vi "MPS_main.vi"() -> ()   [LabVIEW 2021]
uses:
  <vilib>/Analysis/4window.llb/windowTd.ctl
  <vilib>/DAQmx/write.llb/DAQmx Write (Digital Bool 1Line 1Point).vi
  <extravilib>/ChannelInstances/Tag-dbl/Write With Abort.vi
  <vilib>/Utility/file.llb/Write Delimited Spreadsheet (DBL).vi
  MPS_global_variables.vi
  <vilib>/DAQmx/create/channels.llb/DAQmx Create Channel (DO-Digital Output).vi
  <vilib>/DAQmx/miscellaneous.llb/DAQmx Fill In Error Info.vi
  <extravilib>/ChannelInstances/Tag-dbl/Instantiate.vi
  <extravilib>/ChannelInstances/Tag-dbl/Endpoint.vi
  <vilib>/measure/maspectr.llb/FFT Spectrum (Mag-Phase) for 1 Chan.vi
  <extravilib>/ChannelInstances/Tag-dbl.lvlib
  <vilib>/measure/NI_MAPro.lvlib
  <vilib>/Analysis/NI_AALPro.lvlib
  <vilib>/Analysis/NI_AALBase.lvlib
  <vilib>/gmath/NI_Gmath.lvlib
panel:
  out "Last N Drive Amp":dbl[](array[numeric])=[7.800948435870364e-05, 7.800948435870364e-05, 7.800948435870364e-05, 7.800948435870364e-05, 7.800948435870364e-05]
  in  "Divide By val":dbl=2.0
  in  "Divide Mass by X":bool
  in  "Zero Baseline":bool
  out "Waveform Graph":dbl[][](graph)
  out "Sensitivity profile 2":dbl[][](graph)
  out "Recent File Name":string="SP_Fill in name_60_ug_Batch Name"
  in  "name identifier":string="Fill in name"
  in  "Base path":path=path "D:/HumanImagerData/MPS Data"
  out "Meas Drive IMon Val RMS\nCal BMon":dbl=16.19447647785509
  in  "Acq Baseline":bool
  in  "CalcConc":bool
  in  "CalcMass":bool
  in  "Sample MetaData Cluster":T1={"Sample Volume (uL)"=10.0, "Sample Mass (ug)"=60.0, "Sample Conc(mg/mL)"=6.0, "Sample Temperature (C)"=23.0, "Batch Num"=0.0, "Batch Name"="Batch Name", "Solute"="Fe3O4", "Solvent"="Water ", "Sample Description"="Description"}
  in  "TxRx_Params":T2={"sample rate"=2000000.0, "Tx freq"=23809.52380952381, "Tx amp"=0.95, "Tx cycles\nSpectroscopy"=250.0, "Bias amp"=1.4, "Bias freq"=11.904761904761905, "Receive range"=5.0, "Bias Periods\nMagnetometry"=2.0, "Tx Freq Division Factor"=84.0, "Drive Periods per Bias"=2000.0, "TX harmonics"=[47619.04761904762, 71428.57142857142, 95238.09523809524, 119047.61904761905, 142857.14285714284, 166666.66666666666, 190476.19047619047, 214285.7142857143, 238095.2380952381, 261904.7619047619, 285714.2857142857, 309523.8095238095, 333333.3333333333, 357142.85714285716, 380952.38095238095, 404761.90476190473, 428571.4285714286, 452380.95238095237, 476190.4761904762, 500000.0, 523809.5238095238, 547619.0476190476, 571428.5714285714, 595238.0952380953, 619047.619047619, 642857.1428571428, 666666.6666666666, 690476.1904761904, 714285.7142857143, 738095.2380952381, 761904.7619047619, 785714.2857142857, 809523.8095238095, 833333.3333333334, 857142.8571428572, 880952.380952381, 904761.9047619047, 928571.4285714285]} {"TX harmonics" format="%#_6p"; "Tx freq" format="%#_8g"}
  in  "Tab Control 2":enum32{"Motor Params", "Motor Move Control"}(tab)=enum."Motor Move Control"
  out "Motor Dir\nT=Fwd":bool=TRUE
  in  "pulse duration (T/2)":dbl=0.0005 format="%#_13p"
  in  "Motor speed":string(combo)="Full step"
  in  "Sequence to run on start up":string[](array[string])=["Move", "Halt"]
  out "Current Motor State":string="MoveToMax"
  in  "Unsigned Pulses to move":dbl=10.0
  in  "Move-Bed-Back":bool
  in  "Move-Bed-Fwd":bool
  in  "Home then insert sample":bool
  in  "Pulses From Home to Max Sig":dbl=4400.0
  in  "Motor Go Home":bool
  in  "Pulses to move fwd after homing":dbl=150.0 format="%#_13g"
  out "Empty Bore-BMon-Spec":dbl[](array[numeric])
  out "EmptyBoreBaseline_Mag_BMon":dbl[](array[numeric])
  in  "Toggle fan":bool
  out "Amps Drive Peak":dbl=22.902448270514743 format="%#_3p"
  out "EmptyBoreBaseline_Mag":dbl[](array[numeric])
  out "Samples Per Acquisition":dbl=336000.0
  in  "Run Cal BMon":bool
  out "mT/BMon Volt":dbl=145.27846134703603 format="%#_3p"
  out "Meas BMon Val RMS":dbl=0.11147197132801606 format="%#_3p"
  out "Expected mT peak":dbl=10.428171771013478 format="%#_3p"
  in  "Update global variables Button":bool
  in  "stop":bool
  out "current system state":string="Idle"
  out "Main loop has stopped":bool
  in  "Tab Control":T3(tab)
  in  "Tab Control 3":enum32{"Page 1", "Page 2"}(tab)=enum."Page 2"
  out "Mean of mags TF Corr":dbl[](array[numeric])=[4.5198134161737477e-10, 4.705339091228016e-11, 2.4913628541095572e-11, 3.799080385209649e-11, 3.684657264994396e-11, 2.7666013040822994e-11, 2.1562998262072176e-11, 9.35832283593572e-12, 6.785335767128005e-12, 1.618637654777638e-11, 4.453278972759378e-12, 8.695242161562175e-12, 5.505695421570372e-12, 7.599580036290615e-12, 4.816377102414867e-12, 1.3029297120510833e-12, 1.361107900144818e-12, 1.5509807531885633e-13, 1.1494126125683072e-12, 1.8048572256788235e-12, 1.5695940756056345e-12, 4.177554610240691e-12, 5.999424509842453e-12, 4.874978557021519e-12, 9.529122987805845e-12, 5.379691887303521e-12, 9.75617748882951e-12, 1.0753597956189388e-11, 1.383578141946564e-11, 1.3802076818093284e-11, 1.2509628346279071e-11, 1.7443696397243005e-11, 1.9010656363318516e-11, 2.256704924965476e-11, 3.9887752269893355e-11, 3.312089204703278e-11, 2.9142643692279936e-11, 4.5578886589904716e-11, 2.966185216911441e-11, 0.0] format="%#_3p"
  out "mean(FFT) mag":cluster{"Freq array":dbl[], dbl[]}[](graph)
  out "std(FFT)":cluster{"Freq array":dbl[], dbl[]}[](graph)
  out "Std of mags TF Corr":dbl[](array[numeric])=[2.4765666807740003e-10, 2.964765473975954e-11, 1.8138460819953634e-11, 1.2295124978270651e-11, 8.877087369588469e-12, 9.76692294864142e-12, 1.1060107857364228e-11, 5.4800226806312794e-12, 3.1400058412540406e-12, 6.864203903815931e-12, 2.747684195772991e-12, 3.0948587149085473e-12, 2.32071663594191e-12, 2.4779399251558228e-12, 1.8375422203984164e-12, 9.224659898036068e-13, 6.04641015605487e-13, 7.10975452417779e-14, 4.585024773080199e-13, 4.784974514194064e-13, 1.0687637252520008e-12, 1.6948060875352746e-12, 2.7148006011093817e-12, 2.5718695170368923e-12, 4.860185837662061e-12, 2.2698952232635406e-12, 2.837534889875566e-12, 6.3680645161241505e-12, 5.393413394622827e-12, 3.866615680263908e-12, 4.896578402975936e-12, 1.0408434178007631e-11, 1.1521799342350357e-11, 1.2111931519408025e-11, 2.1261630231843856e-11, 2.1498039397344003e-11, 1.6468567943662256e-11, 1.9206279692837516e-11, 1.6162742557341904e-11, 0.0] format="%#_3p"
  out "mean(FFT) Tx Current":cluster{"Freq array":dbl[], dbl[]}(graph)
  out "std(FFT)  Tx Current":cluster{"Freq array":dbl[], dbl[]}(graph)
  in  "Run Sys Ref Meas":bool
  in  "Save SRM":bool
  in  "Spec Tx periods\nto crop SRM":dbl=150.0 format="%#_4p"
  in  "ms delay SRM":u32=5 format="%#.4p"
  in  "Num Avgs SRM":i32=10
  in  "Apply drift \ncorrection?":bool=TRUE
  out "size(s)":i32=4200 format="%.0p"
  out "Loop Num 3":i32=9
  out "Mean_IMon_THD":dbl=0.011152455970515396 format="%#_3p"
  out "MeanIMonTHD_dB":dbl=-39.052589653230974 format="%#_3p"
  in  "Scanner Description":T4={"Scanner Name"="MGH_MIT_MPS", "Hardware description"="Test", "Preamplifier Used"="INA", "Preamp Gain"=9999.0, "Drive Amplifier"="RCF IPS700_CH1", "Bias Amplifier"="RCF IPS700_CH2", "Drive Current Monitor"="Rogowski", "Bias Current Monitor"="ACS-770"}
  in  "Study and Experiment Description":T5={"Study Number"=1, "Study Name"="Particle Testing", "UUID"="B5C626AE-1F0E-494D-B0C0-DF45A2631BD1", "GUI Open Time"="2023-07-01_12-07-36", "Notes"="Dilution Series"}
  out "3f0 over time":cluster{dbl, dbl}(graph)={9.606056730162145e-13, 8.787008379959242e-12}
  out "Rx FFT":cluster{"f0":dbl, "df":dbl, "magnitude":dbl[]}(graph)={"f0"=0.0, "df"=158.7301587301721, "magnitude"=array[6300 elements]}
  in  "Run Spectroscopy":bool
  in  "Stop Spec":bool
  out "Loop Num":i32=9 format="%#.3p"
  in  "Save Spectroscopy":bool
  in  "Max Spec Runs":i32=500
  in  "ms delay":u32=1 format="%#.4p"
  in  "Spec Tx periods\nto crop":dbl=100.0 format="%#_4p"
  out "Spec Time Domain":waveform(dbl)[](graph)=[{"t0"=timestamp(3771075099.535634 s since 1904-01-01), "dt"=4.999999999999579e-07, "Y"=array[159600 elements], "attributes"=variant("NI_ChannelName"=variant(string "H1/ai7"), "NI_UnitDescription"=variant(string "Volts"))}, {"t0"=timestamp(3771075099.535634 s since 1904-01-01), "dt"=4.999999999999579e-07, "Y"=array[159600 elements], "attributes"=variant("NI_ChannelName"=variant(string "H1/ai7"), "NI_UnitDescription"=variant(string "Volts"))}, {"t0"=timestamp(3771075099.535634 s since 1904-01-01), "dt"=4.999999999999579e-07, "Y"=array[159600 elements], "attributes"=variant("NI_ChannelName"=variant(string "H1/ai7"), "NI_UnitDescription"=variant(string "Volts"))}]
  out "f0 over time":dbl(graph)=1.7007410257248368e-10
  out "THD":dbl=0.005520776982623166 format="%#_4p"
  out "Expected mT Spec Drive":dbl=6.10435204788981e-05 format="%#_4p"
  out "mean3f0":dbl=3.4713942019657602e-12 format="%#_3p"
  out "standard deviation 3f0":dbl=1.6525895136355058e-12 format="%#_4p"
  out "meanf0":dbl=1.0516138967766213e-10 format="%#_3p"
  out "standard deviation f0":dbl=4.090729980375604e-11 format="%#_4p"
  out "Ref mT Spec Drive":dbl=7.800948435870364e-05 format="%#_4p"
  in  "UseFeedback":bool
  out "f0 Phase over time":dbl(graph)=-0.927647026653393
  in  "Feedback Avging":dbl=5.0 format="%#_13g"
  out "Relative mT Drive":dbl=0.00016343259278743684 format="%#_3p"
  out "Updated Tx Amp":dbl=0.5023739790026548
  out "Error":dbl=0.0016712299166545819 format="%#_3p"
  in  "Error Gain":dbl=0.1
  out "Langevin":cluster{"Y":dbl[], "Y":dbl[]}[](graph)=[{"Y"=[-3.899866061425817e-05, -3.9231748974479236e-05, -3.9246824870256426e-05, -3.904388830702801e-05, -3.8622939290039456e-05, -3.798845753237372e-05, -3.714641598259823e-05, -3.609830788135816e-05, -3.484562646899217e-05, -3.3398824400567615e-05, -3.17653678589874e-05, -2.9952723026593753e-05, -2.7975822263882995e-05, -2.584511822356924e-05, -2.3569570322071078e-05, -2.1164110918043826e-05, -1.8640685898287753e-05, -1.6012734384739088e-05, -1.3296681970143925e-05, -1.0508954246793974e-05, -7.66448357105398e-06, -4.776709063440463e-06, -1.8620563154459617e-06, 1.0585693748465211e-06, 3.971728887269857e-06, 6.863983101619107e-06, 9.714426719695402e-06, 1.2511113856608338e-05, 1.5237618920418202e-05, 1.7876023083287668e-05, 2.0415873695016075e-05, 2.284223839813179e-05, 2.5137198363318037e-05, 2.7290300939033318e-05, 2.9291093473156727e-05, 3.1124643605919247e-05, 3.278199191982424e-05, 3.425268576098663e-05, 3.553224541833137e-05, 3.661320470851545e-05, 3.7486604212060796e-05, 3.815244392424258e-05, 3.8606244132429925e-05, 3.8842031887654564e-05, 3.885831394862594e-05, 3.8658076782053854e-05, 3.824132038257107e-05, 3.760655150867529e-05, 3.6758249863472383e-05, 3.5703881622719267e-05, 3.444941972643954e-05, 3.300233035134814e-05, 3.1368586438269434e-05, 2.9558640637570703e-05, 2.7584438836498958e-05, 2.545494045026684e-05, 2.3176118421620688e-05, 2.0765891585527157e-05, 1.8246658487001164e-05, 1.5625885307065433e-05, 1.2912531463566184e-05, 1.0126009030398355e-05, 7.282743608825543e-06, 4.3961743274289376e-06, 1.4857132611988467e-06, -1.4337072243640028e-06, -4.3471547637050135e-06, -7.236710518203559e-06, -1.0085948885939363e-05, -1.2881430738303868e-05, -1.560374400091777e-05, -1.8239449545843204e-05, -2.077809471867073e-05, -2.3203253919419743e-05, -2.5499994785286915e-05, -2.7654878190523024e-05, -2.9655958246518067e-05, -3.148979582892112e-05, -3.314892475944235e-05, -3.462438562405869e-05, -3.5905725772938516e-05, -3.69869722656569e-05, -3.786364539834503e-05, -3.853126546745361e-05], "Y"=[5.7665139055820235e-05, 8.02563342374943e-05, 2.3135954141162975e-05, 3.8370395851491655e-05, 7.666887421492822e-08, -1.6353326745701167e-06, -3.131850109735249e-05, -4.252180215784362e-05, -6.681075201303612e-05, -8.354178500796668e-05, -0.00011232913710735343, -0.00011212036199780602, -0.00015658876280484033, -0.0001388647952584951, -0.0001842459865776697, -0.00017643225669247359, -0.00020075124710503323, -0.00020291853502768815, -0.00021791460296951315, -0.00021365035373967857, -0.00023303765092765828, -0.0002161064064262681, -0.0002478914872234107, -0.00022194556056100495, -0.00024165239405261733, -0.00022831141293448037, -0.00023730193869174858, -0.0002282319404163689, -0.00022891465369582039, -0.00022086199509847537, -0.00021075781792146404, -0.00019855575075151182, -0.0001986104750695162, -0.0001784588780601685, -0.00018112303600478357, -0.00018159513469144167, -0.0001503133846049755, -0.00017229903149902393, -0.00012674935866696186, -0.0001344447370080244, -0.00010040371918754682, -0.0001009590608068881, -8.558721246688338e-05, -6.95419396555478e-05, -6.45994581417109e-05, -3.476218814891166e-05, -2.3990356126791314e-05, 1.1960562969286733e-05, 1.1320497334370813e-05, 6.587790071654025e-05, 4.0726279326073945e-05, 8.901605718512913e-05, 8.626069687517241e-05, 8.544329637751575e-05, 0.000135062345200515, 0.00010999614741809734, 0.0001695727606417653, 0.00015403057543677463, 0.0001959948576704691, 0.00017327275872732083, 0.00020990531288118922, 0.0001997518664420034, 0.0002049616944248637, 0.00023545186254814868, 0.00022864323236331527, 0.000242514729569909, 0.00024575451950278513, 0.0002560532643313125, 0.0002406071678831164, 0.0002579897789412676, 0.00024912003641509693, 0.00024186435247545263, 0.0002420067404885037, 0.0002346130180952614, 0.00019875731606227388, 0.00023575156501463713, 0.00017420343163246103, 0.00020669726980396432, 0.00016896358518337585, 0.00017366163827456087, 0.00013257003132153755, 0.0001464291821418053, 9.116412730574912e-05, 0.00011317623992951899]}]
  in  "Normalize to mass?":bool=TRUE
  out "Regression amplitude over time":dbl(graph)=-7.068788164744519e-14
  out "Bed moving":bool=TRUE
  in  "ms delay\nevery Spec":u32=50 format="%#.4p"
  in  "Run in-out spec":bool
  out "Expected mT Spec Drive 2":dbl=3.214000510187691e-05 format="%#_4p"
  out "Drive Imon THD 2":dbl=0.009364497040628524 format="%#_6p"
  in  "Spec drive periods\nto crop_InOut":dbl=10.0 format="%#_4p"
  out "2,3f0 over time":cluster{dbl, dbl}(graph)={6.564821906628785e-12, 3.2258377206728835e-12}
  out "f0 over time 2":dbl(graph)=5.5854646683007315e-12
  out "Loop Num 2":i32=10 format="%.4p"
  out "Spec Time Domain\nInOut":waveform(dbl)[](graph)=[{"t0"=timestamp(3771074868.9554205 s since 1904-01-01), "dt"=4.999999999999579e-07, "Y"=array[167160 elements], "attributes"=variant("NI_ChannelName"=variant(string "H1/ai7"), "NI_UnitDescription"=variant(string "Volts"))}, {"t0"=timestamp(3771074868.9554205 s since 1904-01-01), "dt"=4.999999999999579e-07, "Y"=array[167160 elements], "attributes"=variant("NI_ChannelName"=variant(string "H1/ai7"), "NI_UnitDescription"=variant(string "Volts"))}, {"t0"=timestamp(3771074868.9554205 s since 1904-01-01), "dt"=4.999999999999579e-07, "Y"=array[167160 elements], "attributes"=variant("NI_ChannelName"=variant(string "H1/ai7"), "NI_UnitDescription"=variant(string "Volts"))}]
  out "Rx FFT 2":cluster{"f0":dbl, "df":dbl, "magnitude":dbl[]}(graph)={"f0"=0.0, "df"=99.20634920635754, "magnitude"=[]}
  in  "Num acq per\ncycle":i32=10
  in  "Save Spectroscopy 2":bool
  in  "Number of cycles":i32=3
  in  "Pulses in/out":dbl=1000.0
  out "Run number":i32=66
  in  "Reset Baseline\nEach out cycle":bool
  out "millisecond timer value":u32=1395956284
  out "3f0 Phase  over time":dbl(graph)=1.0359436442159113
  out "Regression\nAmplitudes":dbl[][](array[numeric])=[[1.9436707759750945e-11, -1.1343917863918756e-12, -7.068788164744519e-14, 5.415752111582207e-14, -6.46822386410476e-13, -1.263401147610588e-14, 3.631228154144562e-14, -6.852826969191325e-14, 1.0445245818185798e-13, 8.623406628958938e-14, 8.406623470601816e-14, 9.260549935399976e-14, -5.309780998322236e-14, -4.930122439467233e-14, -5.243411471831613e-14, 2.841726318005815e-14, 1.2631890797003143e-16, -4.3612646781880773e-16, -1.6379094176067293e-14, -1.2042971147936758e-14, 1.5951960147011336e-15, 1.9599758382159657e-14, 5.597126752853182e-14, 7.113562359300652e-14, 1.6077851987506588e-13, -3.662239331827193e-14, -8.540504325781157e-14, -2.25036809302407e-15, 2.569039895005138e-13, 2.3314789177273286e-13, 5.63034120345455e-14, 1.8426210197334996e-13, -1.3033069840030546e-13, -1.583778564751189e-13, 2.6125632161519025e-13, -3.134764146789033e-13, -1.1272253954134242e-13, 5.961280270660638e-13, -6.818142000226762e-13, 0.0], [7.291670843036698e-11, 4.2913802529312405e-12, 1.0740485819641637e-12, 5.766558227927164e-13, -9.378451123543416e-13, 1.857681416825628e-12, -6.529536439773832e-13, 9.47048499966951e-13, 5.788526762951405e-13, 6.573260545221712e-13, 1.8744563857239436e-13, 1.6843328677319332e-13, 5.278970832844011e-13, 2.666350713213874e-13, 1.5653420611863166e-13, 2.318984320042481e-13, 1.209578751436168e-13, 1.1254455152706186e-14, 4.044144966694959e-14, 6.372031849619692e-14, 1.7636004951228526e-13, 2.0729095384551626e-13, 7.158681845833229e-13, 4.0541666084996895e-13, 4.325782866996485e-13, 4.861189337029247e-13, 5.528119056862703e-13, -1.3397687760561724e-14, 1.6663085196229748e-12, 9.133128673606917e-13, 1.188583198760237e-12, 9.904670318662597e-13, 2.336525432468236e-12, 4.3196177522853825e-13, 8.413556533364202e-13, 1.7509439618320136e-12, 2.1753185235436488e-12, 4.1497473932019925e-12, -2.2624426948689035e-12, 0.0], [-1.1660085448916014e-10, -1.825873468631287e-12, 2.0165347043084308e-12, 5.988898236827468e-13, 9.312888379869387e-12, -2.0753950324409236e-12, 3.1287488576156052e-12, -9.278547386049863e-13, -5.971429102969e-13, -4.584603878718662e-13, 8.356751065313785e-13, 5.706511495216728e-13, -5.008886831327364e-13, 7.35060451715737e-14, 3.7669377018327594e-13, -3.26897406189291e-13, -1.5007595644997676e-13, -9.361661233318304e-15, 7.086402821274635e-14, 1.416761052668294e-13, 8.642074181455239e-14, -1.1574432732645524e-14, -1.3653337844925128e-12, -1.7058277209724034e-13, -6.525331295451737e-13, 1.9937792293213593e-13, 3.0828812530702706e-13, 2.357548402730678e-12, -3.066230889504601e-12, 4.769630534776537e-13, -6.565114200201066e-14, 4.112922149112587e-13, -2.985741553610987e-12, 2.932677528590363e-12, 2.3601480992755747e-12, 3.8297667582018487e-13, -8.618648759312713e-13, -7.637526808352155e-12, 1.493948977865726e-11, 0.0], [-7.116406878107296e-11, -1.9073661696394742e-13, 1.9850354248157095e-12, 1.4610339048845079e-12, 1.0404407059609308e-11, -1.739127868292392e-12, 2.402195308412588e-12, -1.8457017228407035e-12, -2.590684078095412e-13, -9.29660567076036e-13, 9.754038129579093e-13, 4.705048225250803e-13, -4.2133794337017297e-13, -6.205324359690596e-14, 4.599916793191991e-13, -3.50801591558906e-13, -1.852159845413742e-13, -8.448036508807536e-15, 8.370291300100184e-14, 1.618709620218298e-13, 2.7606874881986493e-13, -2.8821659853986255e-13, -1.2110184531861104e-12, -4.919701441241681e-13, -1.0623982663079754e-12, -3.0733592226156285e-13, 3.049692180545495e-13, 3.431980433816672e-12, -3.0271708813301673e-12, 2.173755658109109e-12, -6.157263097330314e-13, 1.506656205095852e-12, -3.3691018718074667e-12, 1.4820617684329302e-12, 4.28020535573626e-12, -1.3079396192339172e-12, -2.0012689770682345e-12, -9.692525514919792e-12, 1.5346948618877538e-11, 0.0], [-4.749291960075668e-11, 2.738152410387833e-12, 2.1918693904496736e-12, 1.1648962527292377e-12, 8.766629112012084e-12, -7.124355119799495e-13, 1.0775688606546016e-12, -1.22924981761517e-12, -9.618841588546646e-14, -1.0370575705509043e-12, 5.756718202041955e-13, 1.6812656818124547e-13, -3.0616671707849676e-13, -1.0112014695107697e-13, 4.616721653768675e-13, -2.0962380479331828e-13, -1.5149077244548438e-13, -9.32456629019904e-15, 6.878759381770749e-14, 9.819397238333542e-14, 2.6215563062151254e-13, -3.7139417794922077e-13, -8.594188817178513e-13, -4.925226148231037e-13, -1.1347493491441962e-12, -4.751698396741352e-13, -3.4590504417721613e-14, 2.8683929383599065e-12, -2.20493653630942e-12, 2.206469267268421e-12, -8.928379924564081e-13, 1.105666371149208e-12, -2.7032407970667745e-12, -3.568081241827319e-13, 3.528268725094504e-12, -2.0705548379893737e-12, -3.0477123978006317e-12, -8.102417391264605e-12, 1.0659845157582852e-11, 0.0], [2.2194112211086557e-10, -2.7468376231391876e-12, -5.891659632352866e-12, -2.4957470860281998e-12, -2.7337065147120135e-11, 3.229906665984752e-12, -5.4377671330940274e-12, 3.758663887573186e-12, 7.748291391015066e-13, 2.112455868213224e-12, -2.351030435636221e-12, -9.074890359269495e-13, 1.0957544259643173e-12, 8.504759704525454e-14, -1.3183709479403022e-12, 8.136411332475517e-13, 4.509690818262364e-13, 3.4210434389618746e-14, -2.0062259703504647e-13, -3.582387017730724e-13, -6.464012370137561e-13, 6.870322994279329e-13, 3.3309637815206005e-12, 1.0445556365232997e-12, 3.0326661103262352e-12, 4.886098815460051e-13, -4.219999673469862e-13, -7.703390818100267e-12, 8.100495865345078e-12, -5.0579822013319844e-12, 1.2441681311383626e-12, -2.37732839518592e-12, 8.61002039015351e-12, -3.5400611150767698e-12, -9.520812504156211e-12, 2.8834252081088233e-12, 5.684914178472676e-12, 2.429172788102618e-11, -3.6711315607441186e-11, 0.0]] format="%#_2p"
  out "SNR":dbl[][](array[numeric])=[[0.9582070116899276], [0.7522427763847704], [0.1178470670427011], [0.1365934757539418], [1.3448725822125491], [0.03077784407634847], [0.11903533341122907], [0.3236458616379869], [0.57971188960492], [0.26174946606390154], [0.29324500087384814], [0.5156601261372233], [0.28525568309278365], [0.3075325731354013], [0.5461474731165268], [0.3444171162737258], [0.003344264879309942], [0.06072602546785359], [0.6564047446924404], [0.1863603815821173], [0.018308542752509895], [0.18790719945790002], [0.3575181846800707], [0.3894616036188684], [0.6789428664754115], [0.1334714505747763], [0.22580941341117614], [0.005496158873636038], [0.551735138829809], [0.47487293799614644], [0.10273556302709154], [0.29035804639235707], [0.17534632924835114], [0.18117004683589177], [0.3651831718948387], [0.29382167647731955], [0.10312837858336013], [0.6539244313397603], [0.5407981706132663], [nan]] format="%#_2p"
  in  "Number of \nsaved runs":i32=1 min=1
  out "SNR per ug":dbl[][](array[numeric])=[[0.015970116861498792], [0.012537379606412841], [0.0019641177840450186], [0.002276557929232363], [0.02241454303687582], [0.0005129640679391412], [0.0019839222235204846], [0.005394097693966449], [0.009661864826748667], [0.004362491101065026], [0.004887416681230802], [0.008594335435620389], [0.004754261384879727], [0.005125542885590021], [0.009102457885275446], [0.005740285271228763], [5.573774798849904e-05], [0.0010121004244642265], [0.01094007907820734], [0.003106006359701955], [0.00030514237920849826], [0.003131786657631667], [0.005958636411334511], [0.00649102672698114], [0.011315714441256858], [0.0022245241762462718], [0.003763490223519602], [9.160264789393396e-05], [0.009195585647163483], [0.00791454896660244], [0.001712259383784859], [0.004839300773205951], [0.0029224388208058524], [0.0030195007805981964], [0.006086386198247311], [0.004897027941288659], [0.0017188063097226688], [0.010898740522329338], [0.009013302843554439], [nan]] format="%#_2p"
  in  "Plotted regressor":u16(ring) items=["In vs Out signal", "Constant offset", "Linear drift", "Quadratic drift", "Cubic drift", "Exponential drift"]
  in  "Plotted harmonic \n(3 = 3f0)":i32=3
  out "Most recent amplitude":dbl=-7.068788164744519e-14
  in  "Run Mag":bool
  out "Susceptibility Curves":cluster{"Y":dbl[], "Y":dbl[]}[](graph)
  in  "Save Mag data":bool
  out "Rx Smooth":dbl[](graph)
  out "Sensitivity profile":dbl[][](graph)
  in  "Num Mag Avgs":i32=2 min=1
  out "RunNum":i32=1
  in  "Pulses in/out 2":dbl=1000.0
  in  "ms delay each run":u32=500
  out "Sample Out":bool=TRUE
  out "RxEmptyBore-Mag":waveform(dbl)(graph)={"t0"=timestamp(3771075480.9636745 s since 1904-01-01), "dt"=4.999999999999579e-07, "Y"=array[336000 elements], "attributes"=variant("NI_ChannelName"=variant(string "H1/ai7"), "NI_UnitDescription"=variant(string "Volts"))}
  out "EmptyBoreBaseline_Spec":dbl[](array[numeric])
  out "RxEmptyBore-Spec":dbl[](graph)
  out "Bmon plot":dbl[](graph)
  out "3f0 vs Mass":T6(graph)=[{"Dilution Array\nConc,f0,f3"=[2.0, 1.0, 0.5, 0.25, 0.125, 0.03125, 0.00392, 4.0, 2.0, 2.0, 1.0, 0.5, 0.25, 0.125, 0.0625, 0.0312, 0.0156, 0.00784, 0.00784, 2.0, 1.0, 0.5, 1.0, 0.5, 0.25, 0.125, 0.0625, 0.03125], "Dilution Array\nConc,f0,f3"=[8.445976108256354e-07, 4.222988054128177e-07, 2.1114940270640884e-07, 1.0557470135320442e-07, 5.278735067660221e-08, 1.3196837669150552e-08, 1.6554113172182452e-09, 1.6891952216512707e-06, 8.445976108256354e-07, 8.445976108256354e-07, 4.222988054128177e-07, 2.1114940270640884e-07, 1.0557470135320442e-07, 5.278735067660221e-08, 2.6393675338301105e-08, 1.317572272887991e-08, 6.587861364439955e-09, 3.3108226344364904e-09, 3.3108226344364904e-09, 8.445976108256354e-07, 4.222988054128177e-07, 2.1114940270640884e-07, 4.222988054128177e-07, 2.1114940270640884e-07, 1.0557470135320442e-07, 5.278735067660221e-08, 2.6393675338301105e-08, 1.3196837669150552e-08]}, {"Dilution Array\nConc,f0,f3"=[2.0, 1.0, 0.5, 0.25, 0.125, 0.03125, 0.00392, 4.0, 2.0, 2.0, 1.0, 0.5, 0.25, 0.125, 0.0625, 0.0312, 0.0156, 0.00784, 0.00784, 2.0, 1.0, 0.5, 1.0, 0.5, 0.25, 0.125, 0.0625, 0.03125], "Dilution Array\nConc,f0,f3"=[8.654564201955863e-07, 3.888457243986579e-07, 1.8175578984007196e-07, 1.003944467151888e-07, 4.326222197660144e-08, 1.1797547296422039e-08, 1.581841665406943e-09, 1.6777246169447193e-06, 8.657364297039021e-07, 8.653724510372214e-07, 3.8247844007075894e-07, 1.589503280696296e-07, 9.667718235655813e-08, 4.981226775379863e-08, 2.817177957875589e-08, 1.4846812462359069e-08, 5.347321077082192e-09, 3.726836263683804e-09, 3.5880283461238924e-09, 8.773340342340031e-07, 4.1220973202929997e-07, 1.824870066459054e-07, 4.268310115072778e-07, 1.8946017955254166e-07, 1.240434968362624e-07, 5.316011802759914e-08, 2.80775364006094e-08, 9.18724217005141e-09]}]
  in  "Run DilutionAdd":bool
  in  "ms delay 2":u32=25 format="%#.4p"
  in  "File Name Dilution":string="450ng_Syno"
  out "Expected mT Spec Drive 3":dbl=9.85980807433939 format="%#_4p"
  out "THD 2":dbl=-77.62036234726554 format="%#_6p"
  in  "Spec samples\nto crop 3":dbl=840.0 format="%#_4p"
  in  "Num Dil Series Runs":i32=7
  in  "Clear Dilution Array":bool
  out "r^2":dbl=0.9977469801598665 format="%.4f"
  in  "Delete Last Meas":bool
  out "Dilution Array\nConc,f0,f3":dbl[][](array[numeric])=[[2.0, 8.015906965845593e-06, 8.654564201955863e-07], [1.0, 3.8014401349584595e-06, 3.888457243986579e-07], [0.5, 2.7505781215229744e-06, 1.8175578984007196e-07], [0.25, 1.4298534602411336e-06, 1.003944467151888e-07], [0.125, 1.0890612375135868e-06, 4.326222197660144e-08], [0.03125, 7.748521740995462e-07, 1.1797547296422039e-08], [0.00392, 5.731323027332732e-06, 1.581841665406943e-09], [4.0, 1.3065575131116893e-05, 1.6777246169447193e-06], [2.0, 7.799468791667333e-06, 8.657364297039021e-07], [2.0, 9.669083797019069e-06, 8.653724510372214e-07], [1.0, 3.6527278636967915e-06, 3.8247844007075894e-07], [0.5, 9.05326137733504e-07, 1.589503280696296e-07], [0.25, 2.2151979045769883e-06, 9.667718235655813e-08], [0.125, 5.253565148675961e-07, 4.981226775379863e-08], [0.0625, 1.1506890682533175e-06, 2.817177957875589e-08], [0.0312, 8.239014617114767e-07, 1.4846812462359069e-08], [0.0156, 7.398262739276385e-07, 5.347321077082192e-09], [0.00784, 6.466954115257952e-07, 3.726836263683804e-09], [0.00784, 3.381884494480326e-07, 3.5880283461238924e-09], [2.0, 9.649007743338577e-06, 8.773340342340031e-07], [1.0, 4.4644729979279834e-06, 4.1220973202929997e-07], [0.5, 1.8062663221230199e-06, 1.824870066459054e-07], [1.0, 4.459255500601374e-06, 4.268310115072778e-07], [0.5, 4.682343388000217e-06, 1.8946017955254166e-07], [0.25, 2.265237134878171e-06, 1.240434968362624e-07], [0.125, 1.2321302744093896e-06, 5.316011802759914e-08], [0.0625, 3.184949140969371e-07, 2.80775364006094e-08], [0.03125, 0.00011052586058144889, 9.18724217005141e-09]]
  in  "Save Dilution Array":bool
  # "MPS"
  # "FILE SAVING"
  # "The file will save as:\n[Time stamp]_[MODE]_[name identifier]_[mass]_[Batch name].h5\n\nRemember to update metadata as needed"
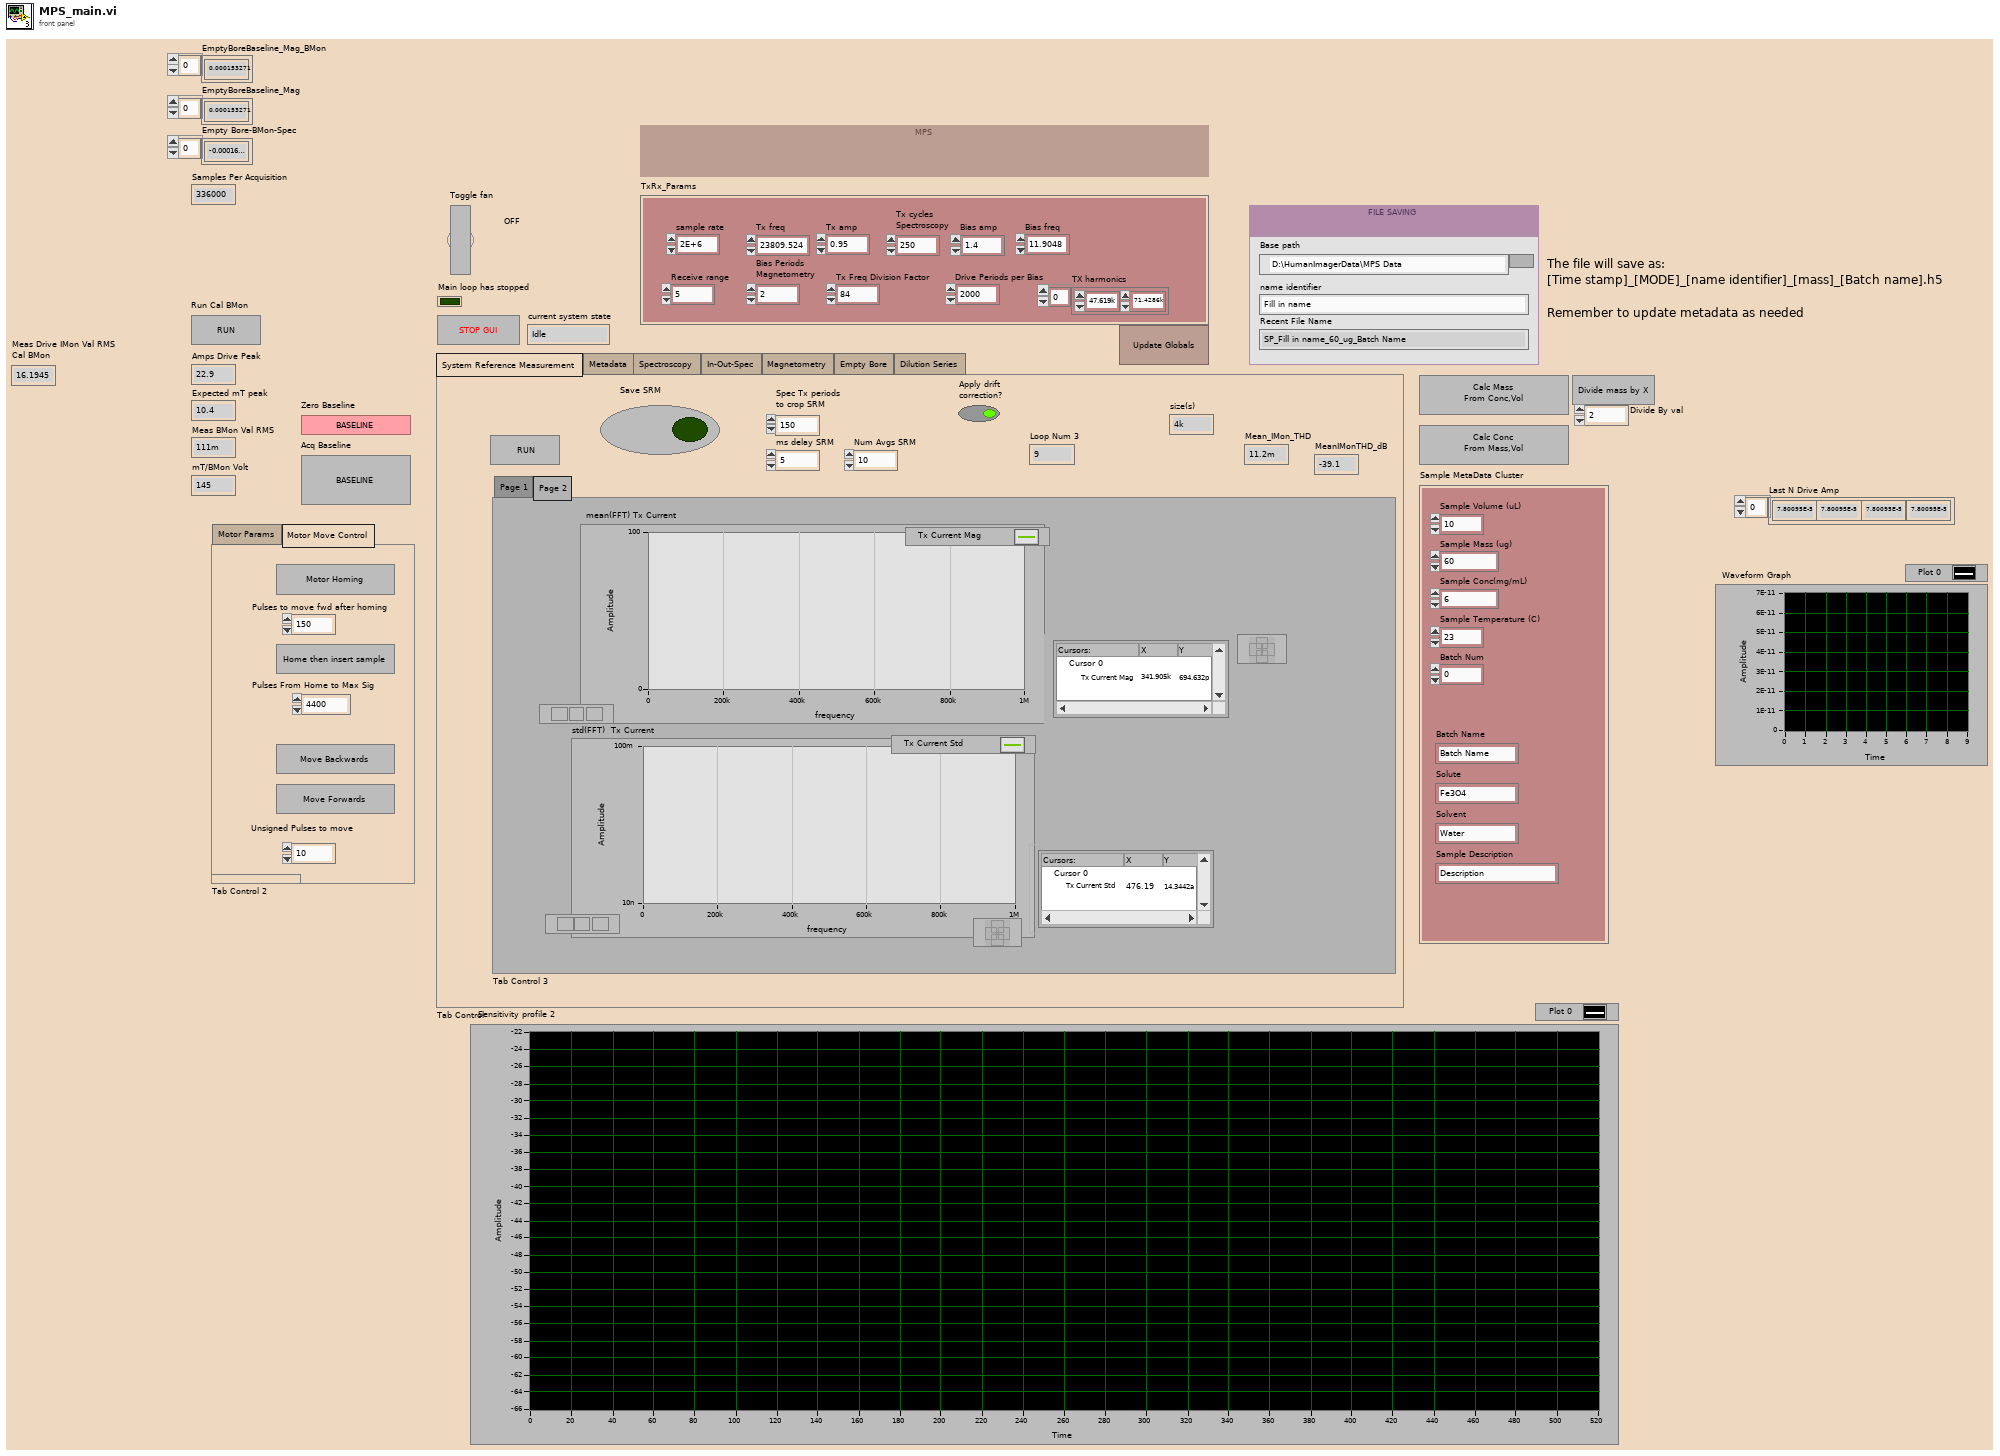
[diagram p1: front panel]
types:
  T1 = cluster{"Sample Volume (uL)":dbl, "Sample Mass (ug)":dbl, "Sample Conc(mg/mL)":dbl, "Sample Temperature (C)":dbl, "Batch Num":dbl, "Batch Name":string, "Solute":string, "Solvent":string, "Sample Description":string}
  T2 = cluster{"sample rate":dbl, "Tx freq":dbl, "Tx amp":dbl, "Tx cycles\nSpectroscopy":dbl, "Bias amp":dbl, "Bias freq":dbl, "Receive range":dbl, "Bias Periods\nMagnetometry":dbl, "Tx Freq Division Factor":dbl, "Drive Periods per Bias":dbl, "TX harmonics":dbl[]}
  T3 = enum32{"System Reference Measurement", "Metadata", "Spectroscopy", "In-Out-Spec", "Magnetometry", "Empty Bore", "Dilution Series"}
  T4 = cluster{"Scanner Name":string, "Hardware description":string, "Preamplifier Used":string, "Preamp Gain":dbl, "Drive Amplifier":string, "Bias Amplifier":string, "Drive Current Monitor":string, "Bias Current Monitor":string}
  T5 = cluster{"Study Number":i64, "Study Name":string, "UUID":string, "GUI Open Time":string, "Notes":string}
  T6 = cluster{"Dilution Array\nConc,f0,f3":dbl[], "Dilution Array\nConc,f0,f3":dbl[]}[]
  T7 = cluster{"Mean of Mags\nTF Corrected":dbl[], "Mean of Phase\nTF Corrected":dbl[], "Std of Mags\nTF Corrected":dbl[], "Std of Phase\nTF Corrected 4":dbl[], "All Mag":dbl[][], "All Phase":dbl[][], "RxFFTMag_AllFreqs":dbl[], "RxFFTPhase_AllFreqs":dbl[], "Std-RxFFT_AllFreqs":dbl[], "Rx_PSD_AllFreqs":dbl[], "Std-Rx_PSD_AllFreqs":dbl[], "TxFFTMag_AllFreqs":dbl[], "TxFFTPhase_AllFreqs":dbl[], "Std-TxFFT_AllFreqs":dbl[], "freqs":dbl[]}
  T8 = cluster{"sample rate":dbl, "Transmit frequency":dbl, "Transmit amplitude":dbl, "sample rate digital out":dbl, "TX cycles":i32, "sample rate DAQ1":dbl, "Receive frequency":dbl, "Receive range":dbl, "TX harmonics":dbl[]}
  T9 = cluster{"Drive IMon":dbl[], "Rx Time Domain":dbl[], "Rx Empty Bore":dbl[], "BMon":dbl[], "Bias IMon":dbl[], "TF-Corr-MagOverTime":dbl[], "Interpolated Rx TF-Mag":dbl[], "Interpolated Rx TF-Phase":dbl[]}
  T10 = cluster{"slope min":dbl, "slope max":dbl, "intercept min":dbl, "intercept max":dbl}
  T11 = cluster{"Sample in_vs_Out":dbl[], "Sample Timing":dbl[]}
  T12 = cluster{"f0":dbl, "df":dbl, "magnitude":dbl[], "phase":dbl[], "PSD":dbl[]}
  T13 = cluster{"TF Corr Rx FFT complex":cluster{"f0":dbl, "df":dbl, "magnitude":dbl[], "phase":dbl[], "PSD":dbl[]}, "output waveform":waveform(dbl)}
  T14 = cluster{dbl[], dbl[], dbl[], cdb[], dbl[], dbl[], dbl[], dbl[], "Freq array":dbl[]}
  T15 = typedef "NI_AALPro.lvlib/windowTd.ctl" = u32
  T16 = typedef "Tag-dbl.lvlib/))Channel.ctl" = refnum<queue>
  T17 = cluster{"Dilution Array\nConc,f0,f3":dbl[], "Best Linear Fit":dbl[]}
  T18 = cluster{"Dilution Array\nConc,f0,f3":dbl[], "Dilution Array\nConc,f0,f3":dbl[]}